vi "Test Update 2.vi"(11 "Test Case In":refnum<class "Camera Tests.lvclass">) -> (0 "error out":errorcluster, 3 "Test Case Out":refnum<class "Camera Tests.lvclass">)   [LabVIEW 2021, in "Camera Tests.lvclass"]
uses:
  Camera Tests.lvclass
  4993e8ee-a06a-463a-9684-69129f64d5ce.vi
  Application Specific/Camera/Camera.lvclass
  Re-use Libraries/Vector 2D/Vector 2D.lvclass
  e086f2d9-95d8-4aa4-9347-c0290e2d8edc.vi
  2d55a890-906c-48cb-a62d-29c0ed2e5d51.vi
  f09cf2b5-a588-4783-9ca3-2cecef7e4928.vi
  63e5ba91-3e82-464b-bdec-192bc4fc123f.vi
  196cb287-c3f0-43e1-8a20-0addf61af9bb.vi
  f4d415ec-62ec-4b9b-b3f1-b0918dc44e12.vi
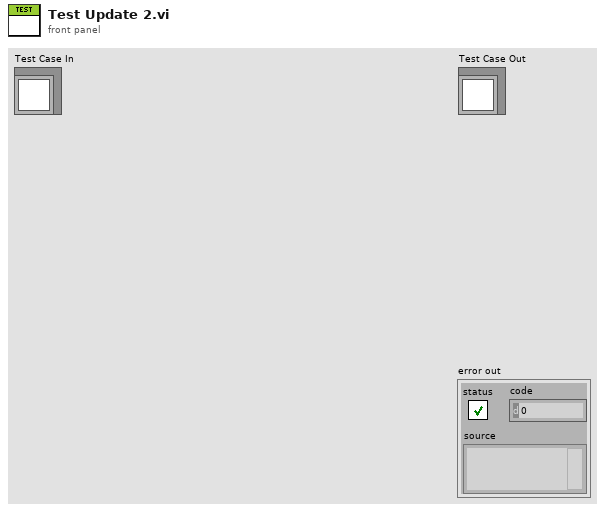
[diagram p1: front panel]
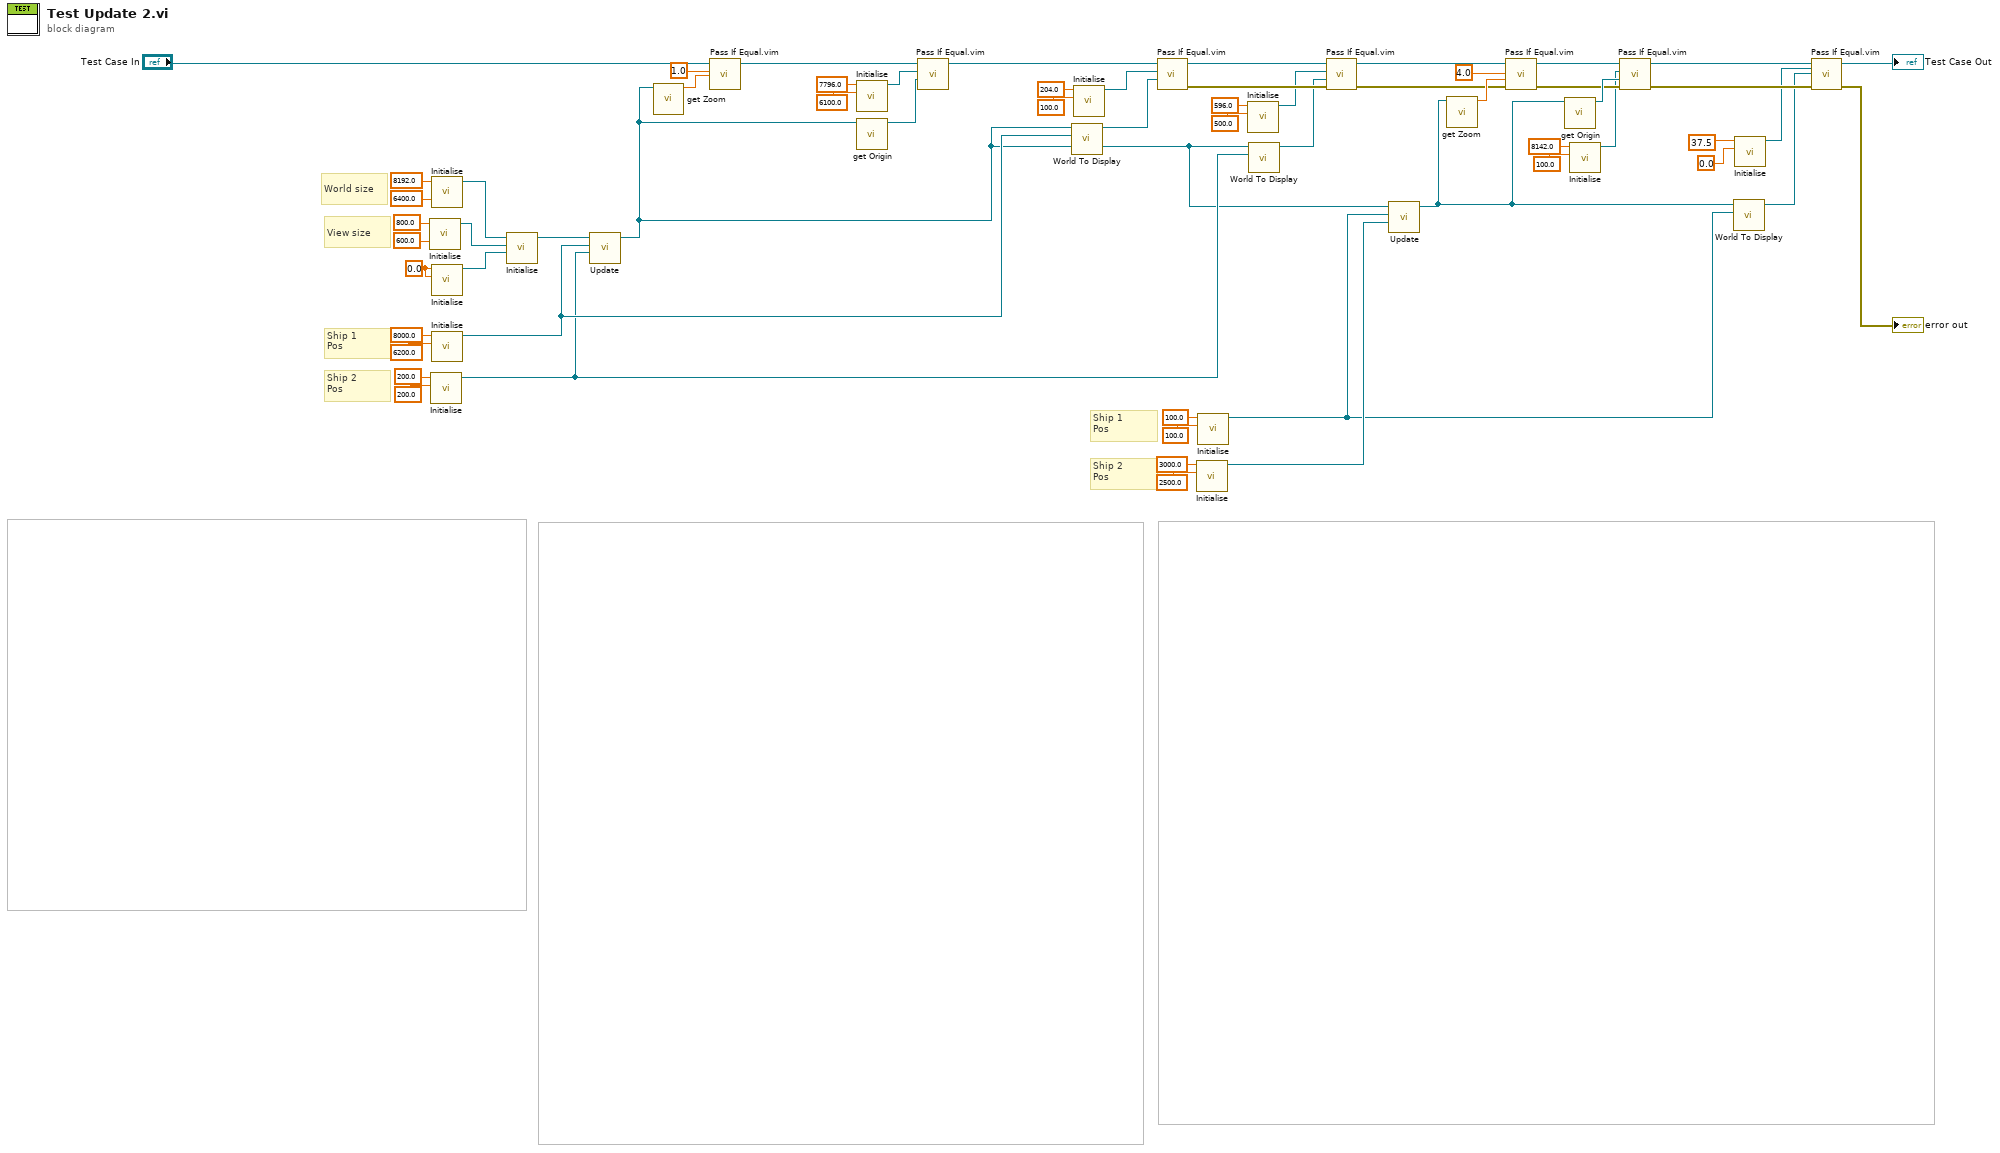
[diagram p0: block diagram]
diagram:
  w56 = sgl 0.0 ("x")
  # "Ship 2\nPos"
  # "Ship 1\nPos"
  # "Ship 2\nPos"
  # "Ship 1\nPos"
  # "View size"
  # "World size"
  n1 = call "Initialise.vi"("y"=sgl 600.0, "x"=sgl 800.0) -> ("Vector 2D out"=w40:refnum<class "Vector 2D.lvclass">)  [unwired: 9 in]
  n2 = call "Initialise.vi"("y"=sgl 200.0, "x"=sgl 200.0) -> ("Vector 2D out"=w33:refnum<class "Vector 2D.lvclass">)  [unwired: 9 in]
  n3 = call "Initialise.vi"("y"=sgl 6400.0, "x"=sgl 8192.0) -> ("Vector 2D out"=w57:refnum<class "Vector 2D.lvclass">)  [unwired: 9 in]
  n4 = call "Initialise.vi"("y"=w56, "x"=w56) -> ("Vector 2D out"=w55:refnum<class "Vector 2D.lvclass">)  [unwired: 9 in]
  n5 = call "Initialise.vi"("y"=sgl 6200.0, "x"=sgl 8000.0) -> ("Vector 2D out"=w47:refnum<class "Vector 2D.lvclass">)  [unwired: 9 in]
  n6 = call "Initialise.vi"("Origin"=w55, "View Size"=w40, "World Size"=w57) -> ("Camera out"=w50:refnum<class "Camera.lvclass">)  [unwired: 8 in]
  n7 = call "Update.vi"("Player 2 Position"=w33, "Player 1 Position"=w47, "Camera in"=w50) -> ("Camera out"=w22:refnum<class "Camera.lvclass">)  [unwired: 8 in]
  n8 = call "get Zoom.vi"("Camera in"=w22) -> ("Zoom Level"=w39:sgl)  [unwired: 10 in]
  n9 = call "Pass If Equal.vim"("Actual"=w39, "Expected"=sgl 1.0 ("Zoom Level"), "LUnit Test Case In"="Test Case In") -> ("LUnit Test Case Out"=w37:refnum<class "Camera Tests.lvclass">)  [unwired: 7 in, 1 out]
  n10 = call "Initialise.vi"("y"=sgl 6100.0, "x"=sgl 7796.0) -> ("Vector 2D out"=w35:refnum<class "Vector 2D.lvclass">)  [unwired: 9 in]
  n11 = call "get Origin.vi"("Camera in"=w22) -> ("Origin"=w34:refnum<class "Vector 2D.lvclass">)  [unwired: 10 in]
  n12 = call "Pass If Equal.vim"("Actual"=w34, "Expected"=w35, "LUnit Test Case In"=w37) -> ("LUnit Test Case Out"=w36:refnum<class "Camera Tests.lvclass">)  [unwired: 7 in, 1 out]
  n13 = call "World To Display.vi"("World Position"=w47, "Camera in"=w22) -> ("Display Position"=w43:refnum<class "Vector 2D.lvclass">)  [unwired: 9 in]
  n14 = call "Initialise.vi"("y"=sgl 100.0, "x"=sgl 204.0) -> ("Vector 2D out"=w44:refnum<class "Vector 2D.lvclass">)  [unwired: 9 in]
  n15 = call "Pass If Equal.vim"("Actual"=w43, "Expected"=w44, "LUnit Test Case In"=w36) -> ("error out"=w31:errorcluster, "LUnit Test Case Out"=w32:refnum<class "Camera Tests.lvclass">)  [unwired: 7 in]
  n16 = call "Initialise.vi"("y"=sgl 2500.0, "x"=sgl 3000.0) -> ("Vector 2D out"=w21:refnum<class "Vector 2D.lvclass">)  [unwired: 9 in]
  n17 = call "Initialise.vi"("y"=sgl 100.0, "x"=sgl 100.0) -> ("Vector 2D out"=w4:refnum<class "Vector 2D.lvclass">)  [unwired: 9 in]
  n18 = call "Initialise.vi"("y"=sgl 500.0, "x"=sgl 596.0) -> ("Vector 2D out"=w27:refnum<class "Vector 2D.lvclass">)  [unwired: 9 in]
  n19 = call "World To Display.vi"("World Position"=w33, "Camera in"=w22) -> ("Display Position"=w28:refnum<class "Vector 2D.lvclass">)  [unwired: 9 in]
  n20 = call "Pass If Equal.vim"("error in (no error)"=w31, "Actual"=w28, "Expected"=w27, "LUnit Test Case In"=w32) -> ("error out"=w13:errorcluster, "LUnit Test Case Out"=w20:refnum<class "Camera Tests.lvclass">)  [unwired: 6 in]
  n21 = call "Update.vi"("Player 2 Position"=w21, "Player 1 Position"=w4, "Camera in"=w22) -> ("Camera out"=w6:refnum<class "Camera.lvclass">)  [unwired: 8 in]
  n22 = call "get Zoom.vi"("Camera in"=w6) -> ("Zoom Level"=w17:sgl)  [unwired: 10 in]
  n23 = call "Pass If Equal.vim"("Delta"=w13, "Actual"=w17, "Expected"=sgl 4.0 ("Zoom Level"), "LUnit Test Case In"=w20) -> ("error out"=w12:errorcluster, "LUnit Test Case Out"=w19:refnum<class "Camera Tests.lvclass">)  [unwired: 6 in]
  n24 = call "get Origin.vi"("Camera in"=w6) -> ("Origin"=w15:refnum<class "Vector 2D.lvclass">)  [unwired: 10 in]
  n25 = call "Initialise.vi"("y"=sgl 100.0, "x"=sgl 8142.0) -> ("Vector 2D out"=w7:refnum<class "Vector 2D.lvclass">)  [unwired: 9 in]
  n26 = call "Pass If Equal.vim"("error in (no error)"=w12, "Actual"=w15, "Expected"=w7, "LUnit Test Case In"=w19) -> ("error out"=w11:errorcluster, "LUnit Test Case Out"=w18:refnum<class "Camera Tests.lvclass">)  [unwired: 6 in]
  n27 = call "World To Display.vi"("World Position"=w4, "Camera in"=w6) -> ("Display Position"=w3:refnum<class "Vector 2D.lvclass">)  [unwired: 9 in]
  n28 = call "Initialise.vi"("y"=sgl 0.0, "x"=sgl 37.5) -> ("Vector 2D out"=w5:refnum<class "Vector 2D.lvclass">)  [unwired: 9 in]
  n29 = call "Pass If Equal.vim"("error in (no error)"=w11, "Actual"=w3, "Expected"=w5, "LUnit Test Case In"=w18) -> ("error out"=→"error out":errorcluster, "LUnit Test Case Out"=→"Test Case Out":refnum<class "Camera Tests.lvclass">)  [unwired: 6 in]
